vi "Dresden R2R Sputter 03.02.2018 IY24.vi"() -> ()   [LabVIEW 2009] (continued)
                                n28839 = case shown="False" w33825 {
                                frame #0 {
                                n28840 = local write "Pc_bv4_auto_set_pressure"(TRUE ("Pc_bv1_auto_set_pressure")) -> ()
                                }
                                frame #1 {
                                }
                                }
                                }
                                frame #1 {
                                }
                                }
                                }
                                frame #6 {
                                n28841 = local read "Semi"() -> (w33831:bool)
                                n28842 = case shown="False" w33831 {
                                frame #0 {
                                n28843 = while {
                                i -> [w33842]
                                stop <- w33833 stop-if-true
                                n28844 = local read "Set_pressure_value 4"() -> (w33837:dbl)
                                n28845 = Greater?(x=w33842, y=300) -> (0:w33835:bool)
                                n28846 = Add(x=1.0, y=w33837) -> (x+y=w33838:dbl)
                                n28847 = Subtract(x=w33837, y=1.0) -> (x-y=w33839:dbl)
                                n28848 = local read "Pressure 4"() -> (w33832:i32)
                                n28849 = In Range and Coerce(upper limit=w33838, x=w33832, lower limit=w33839) -> (In Range?=w33836:bool)  [unwired: 1 out]
                                n28850 = case shown="False" w33836 {
                                tunnel: [FALSE TRUE] -> w33834
                                frame #0 {
                                n28851 = Wait Until Next ms Multiple(millisecond multiple=u32 200) -> ()  [unwired: 1 out]
                                }
                                frame #1 {
                                }
                                }
                                n28852 = Or(x=w33834, y=w33835) -> (x .or. y?=w33833:bool)
                                }
                                }
                                frame #1 {
                                }
                                }
                                }
                                frame #7 {
                                n28853 = local read "Semi"() -> (w33847:bool)
                                n28854 = case shown="False" w33847 {
                                frame #0 {
                                n28855 = local read "Set_pressure_value 4"() -> (w33850:dbl)
                                n28856 = Add(x=1.0, y=w33850) -> (x+y=w33851:dbl)
                                n28857 = Subtract(x=w33850, y=1.0) -> (x-y=w33852:dbl)
                                n28858 = local read "Pressure 4"() -> (w33848:i32)
                                n28859 = In Range and Coerce(upper limit=w33851, x=w33848, lower limit=w33852) -> (In Range?=w33849:bool)  [unwired: 1 out]
                                n28860 = case shown="False" w33849 {
                                frame #0 {
                                n28861 = local write "Semi"(TRUE ("Semi")) -> ()
                                n28862 = local write "Error Message"("Coating Pressure could not be adjusted !" ("Error Message")) -> ()
                                }
                                frame #1 {
                                }
                                }
                                }
                                frame #1 {
                                }
                                }
                                }
                                }
                                }
                                frame #1 {
                                }
                                }
                                }
                                frame #1 {
                                n28863 = local read "Semi"() -> (w33857:bool)
                                n28864 = case shown="False" w33857 {
                                frame #0 {
                                n28865 = local write "SDC1 9"(TRUE ("SDC1 9")) -> ()
                                n28866 = Wait (ms)(milliseconds to wait=u32 1000) -> ()  [unwired: 1 out]
                                }
                                frame #1 {
                                }
                                }
                                }
                                }
                                }
                                }
                                }
                                frame #1 {
                                }
                                }
                                }
                                frame #11 {
                                n28867 = local read "Semi"() -> (w33860:bool)
                                n28868 = case shown="False" w33860 {
                                frame #0 {
                                n28869 = local write "Start_roll"(TRUE ("Start_roll")) -> ()
                                n28870 = Wait (ms)(milliseconds to wait=u32 300) -> ()  [unwired: 1 out]
                                }
                                frame #1 {
                                }
                                }
                                }
                                frame #12 {
                                n28871 = local read "Semi"() -> (w33863:bool)
                                n28872 = case shown="False" w33863 {
                                frame #0 {
                                n28873 = stacked-sequence {
                                frame #0 {
                                n28874 = local read "R Single RF Step1 Coating Power Active"() -> (w33864:bool)
                                n28875 = case shown="True" w33864 {
                                frame #0 {
                                }
                                frame #1 {
                                n28876 = while {
                                stop <- w33866 stop-if-true
                                n28877 = local read "R Single RF Interval length"() -> (w33870:dbl)
                                n28878 = local read "Actual Length"() -> (w33869:dbl)
                                n28879 = Greater Or Equal?(x=w33869, y=w33870) -> (x >= y?=w33868:bool)
                                n28880 = local read "Semi"() -> (w33867:bool)
                                n28881 = Or(x=w33868, y=w33867) -> (x .or. y?=w33866:bool)
                                n28882 = Wait Until Next ms Multiple(millisecond multiple=u32 300) -> ()  [unwired: 1 out]
                                }
                                }
                                }
                                }
                                frame #1 {
                                n28883 = local read "R Single RF Step2 Coating Power Active"() -> (w33871:bool)
                                n28884 = case shown="True" w33871 {
                                frame #0 {
                                }
                                frame #1 {
                                n28885 = stacked-sequence {
                                frame #0 {
                                n28886 = local read "Semi"() -> (w33872:bool)
                                n28887 = case shown="False" w33872 {
                                frame #0 {
                                n28888 = local read "R Single RF Step2 Coating Power"() -> (w33874:dbl)
                                n28889 = Wait (ms)(milliseconds to wait=u32 200) -> ()  [unwired: 1 out]
                                n28890 = local write "RF_forward_power_1"(w33874) -> ()
                                }
                                frame #1 {
                                }
                                }
                                }
                                frame #1 {
                                n28891 = local read "Semi"() -> (w33875:bool)
                                n28892 = case shown="False" w33875 {
                                frame #0 {
                                n28893 = local write "RF set auto"(TRUE ("Dc_auto_set")) -> ()
                                }
                                frame #1 {
                                }
                                }
                                }
                                frame #2 {
                                n28894 = while {
                                stop <- w33881 stop-if-true
                                n28895 = local read "R Single RF Interval length"() -> (w33880:dbl)
                                n28896 = local read "Actual Length"() -> (w33884:dbl)
                                n28897 = Multiply(x=w33880, y=2.0) -> (x*y=w33878:dbl)
                                n28898 = Greater Or Equal?(x=w33884, y=w33878) -> (x >= y?=w33883:bool)
                                n28899 = local read "Semi"() -> (w33882:bool)
                                n28900 = Or(x=w33883, y=w33882) -> (x .or. y?=w33881:bool)
                                n28901 = Wait Until Next ms Multiple(millisecond multiple=u32 300) -> ()  [unwired: 1 out]
                                }
                                }
                                }
                                }
                                }
                                }
                                frame #2 {
                                n28902 = local read "R Single RF Step3 Coating Power Active"() -> (w33885:bool)
                                n28903 = case shown="True" w33885 {
                                frame #0 {
                                }
                                frame #1 {
                                n28904 = stacked-sequence {
                                frame #0 {
                                n28905 = local read "Semi"() -> (w33886:bool)
                                n28906 = case shown="False" w33886 {
                                frame #0 {
                                n28907 = local read "R Single RF Step3 Coating Power"() -> (w33888:dbl)
                                n28908 = Wait (ms)(milliseconds to wait=u32 200) -> ()  [unwired: 1 out]
                                n28909 = local write "RF_forward_power_1"(w33888) -> ()
                                }
                                frame #1 {
                                }
                                }
                                }
                                frame #1 {
                                n28910 = local read "Semi"() -> (w33889:bool)
                                n28911 = case shown="False" w33889 {
                                frame #0 {
                                n28912 = local write "RF set auto"(TRUE ("Dc_auto_set")) -> ()
                                }
                                frame #1 {
                                }
                                }
                                }
                                frame #2 {
                                n28913 = while {
                                stop <- w33895 stop-if-true
                                n28914 = local read "R Single RF Interval length"() -> (w33894:dbl)
                                n28915 = local read "Actual Length"() -> (w33898:dbl)
                                n28916 = Multiply(x=w33894, y=3.0) -> (x*y=w33892:dbl)
                                n28917 = Greater Or Equal?(x=w33898, y=w33892) -> (x >= y?=w33897:bool)
                                n28918 = local read "Semi"() -> (w33896:bool)
                                n28919 = Or(x=w33897, y=w33896) -> (x .or. y?=w33895:bool)
                                n28920 = Wait Until Next ms Multiple(millisecond multiple=u32 300) -> ()  [unwired: 1 out]
                                }
                                }
                                }
                                }
                                }
                                }
                                frame #3 {
                                n28921 = local read "R Single RF Step4 Coating Power Active"() -> (w33899:bool)
                                n28922 = case shown="True" w33899 {
                                frame #0 {
                                }
                                frame #1 {
                                n28923 = stacked-sequence {
                                frame #0 {
                                n28924 = local read "Semi"() -> (w33900:bool)
                                n28925 = case shown="False" w33900 {
                                frame #0 {
                                n28926 = local read "R Single RF Step4 Coating Power"() -> (w33902:dbl)
                                n28927 = Wait (ms)(milliseconds to wait=u32 200) -> ()  [unwired: 1 out]
                                n28928 = local write "RF_forward_power_1"(w33902) -> ()
                                }
                                frame #1 {
                                }
                                }
                                }
                                frame #1 {
                                n28929 = local read "Semi"() -> (w33903:bool)
                                n28930 = case shown="False" w33903 {
                                frame #0 {
                                n28931 = local write "RF set auto"(TRUE ("Dc_auto_set")) -> ()
                                }
                                frame #1 {
                                }
                                }
                                }
                                frame #2 {
                                n28932 = while {
                                stop <- w33909 stop-if-true
                                n28933 = local read "R Single RF Interval length"() -> (w33908:dbl)
                                n28934 = local read "Actual Length"() -> (w33912:dbl)
                                n28935 = Multiply(x=w33908, y=4.0) -> (x*y=w33906:dbl)
                                n28936 = Greater Or Equal?(x=w33912, y=w33906) -> (x >= y?=w33911:bool)
                                n28937 = local read "Semi"() -> (w33910:bool)
                                n28938 = Or(x=w33911, y=w33910) -> (x .or. y?=w33909:bool)
                                n28939 = Wait Until Next ms Multiple(millisecond multiple=u32 300) -> ()  [unwired: 1 out]
                                }
                                }
                                }
                                }
                                }
                                }
                                frame #4 {
                                n28940 = local read "R Single RF Step5 Coating Power Active"() -> (w33913:bool)
                                n28941 = case shown="True" w33913 {
                                frame #0 {
                                }
                                frame #1 {
                                n28942 = stacked-sequence {
                                frame #0 {
                                n28943 = local read "Semi"() -> (w33914:bool)
                                n28944 = case shown="False" w33914 {
                                frame #0 {
                                n28945 = local read "R Single RF Step5 Coating Power"() -> (w33916:dbl)
                                n28946 = Wait (ms)(milliseconds to wait=u32 200) -> ()  [unwired: 1 out]
                                n28947 = local write "RF_forward_power_1"(w33916) -> ()
                                }
                                frame #1 {
                                }
                                }
                                }
                                frame #1 {
                                n28948 = local read "Semi"() -> (w33917:bool)
                                n28949 = case shown="False" w33917 {
                                frame #0 {
                                n28950 = local write "RF set auto"(TRUE ("Dc_auto_set")) -> ()
                                }
                                frame #1 {
                                }
                                }
                                }
                                frame #2 {
                                n28951 = while {
                                stop <- w33923 stop-if-true
                                n28952 = local read "R Single RF Interval length"() -> (w33922:dbl)
                                n28953 = local read "Actual Length"() -> (w33926:dbl)
                                n28954 = Multiply(x=w33922, y=5.0) -> (x*y=w33920:dbl)
                                n28955 = Greater Or Equal?(x=w33926, y=w33920) -> (x >= y?=w33925:bool)
                                n28956 = local read "Semi"() -> (w33924:bool)
                                n28957 = Or(x=w33925, y=w33924) -> (x .or. y?=w33923:bool)
                                n28958 = Wait Until Next ms Multiple(millisecond multiple=u32 300) -> ()  [unwired: 1 out]
                                }
                                }
                                }
                                }
                                }
                                }
                                }
                                }
                                frame #1 {
                                }
                                }
                                }
                                frame #13 {
                                n28959 = local read "Semi"() -> (w33927:bool)
                                n28960 = case shown="False" w33927 {
                                frame #0 {
                                n28961 = local write "SDC1 13b"(TRUE ("SDC1 13b")) -> ()
                                n28962 = Wait (ms)(milliseconds to wait=u32 1000) -> ()  [unwired: 1 out]
                                }
                                frame #1 {
                                }
                                }
                                }
                                }
                                }
                                frame #1 {
                                }
                                }
                                }
                                frame #17 {
                                # "encoder info  add to other web selection"
                                n28963 = stacked-sequence {
                                frame #0 {
                                n28964 = local read "Semi"() -> (w33930:bool)
                                n28965 = case shown="False" w33930 {
                                frame #0 {
                                # "salinim hareketi"
                                n28966 = local read "R_Web_selection"() -> (w33931:enum32{"Web", "Other"})
                                n28967 = case shown="\"Other\"" w33931 {
                                frame #0 {
                                # "TC -ROLL"
                                }
                                frame #1 {
                                n28968 = disable-structure shown="Disabled" {
                                frame #0 {
                                # "OTHER"
                                n28969 = local read "Semi"() -> (w33932:bool)
                                n28970 = case shown="False" w33932 {
                                frame #0 {
                                n28971 = stacked-sequence {
                                frame #0 {
                                n28972 = local read "Semi"() -> (w33933:bool)
                                n28973 = case shown="False" w33933 {
                                frame #0 {
                                n28974 = stacked-sequence {
                                frame #0 {
                                n28975 = local read "Semi"() -> (w33934:bool)
                                n28976 = case shown="False" w33934 {
                                frame #0 {
                                n28977 = while {
                                i -> [w33937]
                                stop <- w33938 stop-if-true
                                n28978 = Greater?(x=w33937, y=300) -> (0:w33935:bool)
                                n28979 = case shown="True" w33935 {
                                frame #0 {
                                }
                                frame #1 {
                                n28980 = local write "Semi"(TRUE ("Semi")) -> ()
                                }
                                }
                                n28981 = local read "RC_13"() -> (w33941:bool)
                                n28982 = case shown="False" w33941 {
                                tunnel: [FALSE ("ch2_1") TRUE ("ch2_1")] -> w33940
                                frame #0 {
                                n28983 = local write "Routine_check_transfer"(TRUE ("ch2_1")) -> ()
                                n28984 = Wait Until Next ms Multiple(millisecond multiple=u32 1000) -> ()  [unwired: 1 out]
                                }
                                frame #1 {
                                }
                                }
                                n28985 = local read "Semi"() -> (w33939:bool)
                                n28986 = Or(x=w33940, y=w33939) -> (x .or. y?=w33938:bool)
                                }
                                }
                                frame #1 {
                                }
                                }
                                }
                                frame #1 {
                                n28987 = local read "Semi"() -> (w33947:bool)
                                n28988 = case shown="False" w33947 {
                                frame #0 {
                                n28989 = while {
                                i -> [w33954]
                                stop <- w33949 stop-if-true
                                n28990 = Greater?(x=w33954, y=100) -> (0:w33952:bool)
                                n28991 = case shown="True" w33952 {
                                frame #0 {
                                }
                                frame #1 {
                                n28992 = local write "Error Message"("Transfer process was cancelled.\nPlease check GV connections." ("Error Message")) -> ()
                                n28993 = local write "Semi"(TRUE ("Semi")) -> ()
                                }
                                }
                                n28994 = local read "Ch1_Trns_interlock_di"() -> (w33948:bool)
                                n28995 = case shown="False" w33948 {
                                tunnel: [w33956 TRUE] -> w33951
                                frame #0 {
                                n28996 = local read "Ch1_TGV_control_di"() -> (w33955:bool)
                                n28997 = case shown="False" w33955 {
                                tunnel: [FALSE TRUE] -> w33956
                                frame #0 {
                                n28998 = Wait Until Next ms Multiple(millisecond multiple=u32 50) -> ()  [unwired: 1 out]
                                n28999 = local write "Ch1_TGV_control_do"(TRUE ("Ch1_pet_cool_up_do")) -> ()
                                }
                                frame #1 {
                                }
                                }
                                }
                                frame #1 {
                                }
                                }
                                n29000 = local read "Semi"() -> (w33950:bool)
                                n29001 = Or(x=w33951, y=w33950) -> (x .or. y?=w33949:bool)
                                }
                                }
                                frame #1 {
                                }
                                }
                                }
                                frame #2 {
                                n29002 = local read "Semi"() -> (w33964:bool)
                                n29003 = case shown="False" w33964 {
                                frame #0 {
                                n29004 = while {
                                i -> [w33971]
                                stop <- w33966 stop-if-true
                                n29005 = Greater?(x=w33971, y=100) -> (0:w33969:bool)
                                n29006 = case shown="True" w33969 {
                                frame #0 {
                                }
                                frame #1 {
                                n29007 = local write "Error Message"("Transfer process was cancelled.\nPlease check GV connections." ("Error Message")) -> ()
                                n29008 = local write "Semi"(TRUE ("Semi")) -> ()
                                }
                                }
                                n29009 = local read "Ch2_Trns_interlock_di"() -> (w33965:bool)
                                n29010 = case shown="False" w33965 {
                                tunnel: [w33973 TRUE] -> w33968
                                frame #0 {
                                n29011 = local read "Ch2_TGV_control_di"() -> (w33972:bool)
                                n29012 = case shown="False" w33972 {
                                tunnel: [FALSE TRUE] -> w33973
                                frame #0 {
                                n29013 = Wait Until Next ms Multiple(millisecond multiple=u32 50) -> ()  [unwired: 1 out]
                                n29014 = local write "Ch2_TGV_control_do"(TRUE ("Ch1_pet_cool_up_do")) -> ()
                                }
                                frame #1 {
                                }
                                }
                                }
                                frame #1 {
                                }
                                }
                                n29015 = local read "Semi"() -> (w33967:bool)
                                n29016 = Or(x=w33968, y=w33967) -> (x .or. y?=w33966:bool)
                                }
                                }
                                frame #1 {
                                }
                                }
                                }
                                frame #3 {
                                n29017 = local read "Semi"() -> (w33981:bool)
                                n29018 = case shown="False" w33981 {
                                frame #0 {
                                n29019 = while {
                                i -> [w33988]
                                stop <- w33983 stop-if-true
                                n29020 = Greater?(x=w33988, y=100) -> (0:w33986:bool)
                                n29021 = case shown="True" w33986 {
                                frame #0 {
                                }
                                frame #1 {
                                n29022 = local write "Error Message"("Transfer process was cancelled.\nPlease check GV connections." ("Error Message")) -> ()
                                n29023 = local write "Semi"(TRUE ("Semi")) -> ()
                                }
                                }
                                n29024 = local read "Ch3_Trns_interlock_di"() -> (w33982:bool)
                                n29025 = case shown="False" w33982 {
                                tunnel: [w33990 TRUE] -> w33985
                                frame #0 {
                                n29026 = local read "Ch3_TGV_control_di"() -> (w33989:bool)
                                n29027 = case shown="False" w33989 {
                                tunnel: [FALSE TRUE] -> w33990
                                frame #0 {
                                n29028 = Wait Until Next ms Multiple(millisecond multiple=u32 50) -> ()  [unwired: 1 out]
                                n29029 = local write "Ch3_TGV_control_do"(TRUE ("Ch1_pet_cool_up_do")) -> ()
                                }
                                frame #1 {
                                }
                                }
                                }
                                frame #1 {
                                }
                                }
                                n29030 = local read "Semi"() -> (w33984:bool)
                                n29031 = Or(x=w33985, y=w33984) -> (x .or. y?=w33983:bool)
                                }
                                }
                                frame #1 {
                                }
                                }
                                }
                                frame #4 {
                                n29032 = local read "Semi"() -> (w33998:bool)
                                n29033 = case shown="False" w33998 {
                                frame #0 {
                                n29034 = while {
                                i -> [w34005]
                                stop <- w34000 stop-if-true
                                n29035 = Greater?(x=w34005, y=100) -> (0:w34003:bool)
                                n29036 = case shown="True" w34003 {
                                frame #0 {
                                }
                                frame #1 {
                                n29037 = local write "Error Message"("Transfer process was cancelled.\nPlease check GV connections." ("Error Message")) -> ()
                                n29038 = local write "Semi"(TRUE ("Semi")) -> ()
                                }
                                }
                                n29039 = local read "Ch3_Trns_interlock_di"() -> (w33999:bool)
                                n29040 = case shown="False" w33999 {
                                tunnel: [w34007 TRUE] -> w34002
                                frame #0 {
                                n29041 = local read "Ch3_TGV_control_di"() -> (w34006:bool)
                                n29042 = case shown="False" w34006 {
                                tunnel: [FALSE TRUE] -> w34007
                                frame #0 {
                                n29043 = Wait Until Next ms Multiple(millisecond multiple=u32 50) -> ()  [unwired: 1 out]
                                n29044 = local write "Ch3_TGV_control_do"(TRUE ("Ch1_pet_cool_up_do")) -> ()
                                }
                                frame #1 {
                                }
                                }
                                }
                                frame #1 {
                                }
                                }
                                n29045 = local read "Semi"() -> (w34001:bool)
                                n29046 = Or(x=w34002, y=w34001) -> (x .or. y?=w34000:bool)
                                }
                                }
                                frame #1 {
                                }
                                }
                                }
                                frame #5 {
                                n29047 = local read "Semi"() -> (w34015:bool)
                                n29048 = case shown="False" w34015 {
                                frame #0 {
                                n29049 = while {
                                i -> [w34018]
                                stop <- w34019 stop-if-true
                                n29050 = Greater?(x=w34018, y=50) -> (0:w34016:bool)
                                n29051 = case shown="True" w34016 {
                                frame #0 {
                                }
                                frame #1 {
                                n29052 = local write "Error Message"("Transfer process was\ncancelled.Please check right slow sensor." ("Error Message")) -> ()
                                n29053 = local write "Semi"(TRUE ("Semi")) -> ()
                                }
                                }
                                n29054 = local read "Cnt_Right_slow_di"() -> (w34022:bool)
                                n29055 = case shown="False" w34022 {
                                tunnel: [FALSE ("Ch1_pet_cool_up_do") TRUE ("Ch1_pet_cool_up_do")] -> w34021
                                frame #0 {
                                n29056 = local write "Cnt_Right_slow_do"(TRUE ("Ch1_pet_cool_up_do")) -> ()
                                n29057 = Wait Until Next ms Multiple(millisecond multiple=u32 200) -> ()  [unwired: 1 out]
                                }
                                frame #1 {
                                }
                                }
                                n29058 = local read "Semi"() -> (w34020:bool)
                                n29059 = Or(x=w34021, y=w34020) -> (x .or. y?=w34019:bool)
                                }
                                }
                                frame #1 {
                                }
                                }
                                }
                                frame #6 {
                                n29060 = local read "Semi"() -> (w34029:bool)
                                n29061 = case shown="False" w34029 {
                                frame #0 {
                                n29062 = while {
                                i -> [w34030]
                                stop <- w34034 stop-if-true
                                n29063 = Greater?(x=w34030, y=50) -> (0:w34032:bool)
                                n29064 = case shown="True" w34032 {
                                frame #0 {
                                }
                                frame #1 {
                                n29065 = local write "Error Message"("Transfer process was\ncancelled.Please check right limit sensor." ("Error Message")) -> ()
                                n29066 = local write "Semi"(TRUE ("Semi")) -> ()
                                }
                                }
                                n29067 = local read "Cnt_Right_limit_di"() -> (w34036:bool)
                                n29068 = case shown="False" w34036 {
                                tunnel: [FALSE ("Ch1_pet_cool_up_do") TRUE ("Ch1_pet_cool_up_do")] -> w34035
                                frame #0 {
                                n29069 = local write "Cnt_Right_limit_do"(TRUE ("Ch1_pet_cool_up_do")) -> ()
                                n29070 = Wait Until Next ms Multiple(millisecond multiple=u32 200) -> ()  [unwired: 1 out]
                                }
                                frame #1 {
                                }
                                }
                                n29071 = local read "Semi"() -> (w34033:bool)
                                n29072 = Or(x=w34035, y=w34033) -> (x .or. y?=w34034:bool)
                                }
                                }
                                frame #1 {
                                }
                                }
                                }
                                frame #7 {
                                n29073 = local read "Semi"() -> (w34043:bool)
                                n29074 = case shown="False" w34043 {
                                frame #0 {
                                n29075 = while {
                                i -> [w34046]
                                stop <- w34047 stop-if-true
                                n29076 = Greater?(x=w34046, y=50) -> (0:w34044:bool)
                                n29077 = case shown="True" w34044 {
                                frame #0 {
                                }
                                frame #1 {
                                n29078 = local write "Error Message"("Transfer process was\ncancelled.Please check left slow sensor." ("Error Message")) -> ()
                                n29079 = local write "Semi"(TRUE ("Semi")) -> ()
                                }
                                }
                                n29080 = local read "Cnt_Left_slow_di"() -> (w34050:bool)
                                n29081 = case shown="False" w34050 {
                                tunnel: [FALSE ("Ch1_pet_cool_up_do") TRUE ("Ch1_pet_cool_up_do")] -> w34049
                                frame #0 {
                                n29082 = local write "Cnt_Left_slow_do"(TRUE ("Ch1_pet_cool_up_do")) -> ()
                                n29083 = Wait Until Next ms Multiple(millisecond multiple=u32 200) -> ()  [unwired: 1 out]
                                }
                                frame #1 {
                                }
                                }
                                n29084 = local read "Semi"() -> (w34048:bool)
                                n29085 = Or(x=w34049, y=w34048) -> (x .or. y?=w34047:bool)
                                }
                                }
                                frame #1 {
                                }
                                }
                                }
                                frame #8 {
                                n29086 = local read "Semi"() -> (w34057:bool)
                                n29087 = case shown="False" w34057 {
                                frame #0 {
                                n29088 = while {
                                i -> [w34058]
                                stop <- w34062 stop-if-true
                                n29089 = Greater?(x=w34058, y=50) -> (0:w34060:bool)
                                n29090 = case shown="True" w34060 {
                                frame #0 {
                                }
                                frame #1 {
                                n29091 = local write "Error Message"("Transfer process was\ncancelled.Please check left limit sensor." ("Error Message")) -> ()
                                n29092 = local write "Semi"(TRUE ("Semi")) -> ()
                                }
                                }
                                n29093 = local read "Cnt_Left_limit_di"() -> (w34064:bool)
                                n29094 = case shown="False" w34064 {
                                tunnel: [FALSE ("Ch1_pet_cool_up_do") TRUE ("Ch1_pet_cool_up_do")] -> w34063
                                frame #0 {
                                n29095 = local write "Cnt_Left_limit_do"(TRUE ("Ch1_pet_cool_up_do")) -> ()
                                n29096 = Wait Until Next ms Multiple(millisecond multiple=u32 200) -> ()  [unwired: 1 out]
                                }
                                frame #1 {
                                }
                                }
                                n29097 = local read "Semi"() -> (w34061:bool)
                                n29098 = Or(x=w34063, y=w34061) -> (x .or. y?=w34062:bool)
                                }
                                }
                                frame #1 {
                                }
                                }
                                }
                                }
                                }
                                frame #1 {
                                }
                                }
                                }
                                frame #1 {
                                n29099 = local read "Semi"() -> (w34071:bool)
                                n29100 = case shown="False" w34071 {
                                frame #0 {
                                n29101 = while {
                                i -> [w34077]
                                stop <- w34074 stop-if-true
                                n29102 = Greater?(x=w34077, y=50) -> (0:w34076:bool)
                                n29103 = case shown="True" w34076 {
                                frame #0 {
                                }
                                frame #1 {
                                n29104 = local write "Error Message"("" ("Error Message")) -> ()
                                n29105 = local write "Semi"(TRUE ("Semi")) -> ()
                                }
                                }
                                n29106 = local read "Casette_servo_start/stop_di"() -> (w34073:bool)
                                n29107 = case shown="False" w34073 {
                                tunnel: [FALSE TRUE] -> w34072
                                frame #0 {
                                n29108 = local write "Casette_servo_start/stop_do"(TRUE ("Casette_servo_left_direction_do")) -> ()
                                n29109 = Wait Until Next ms Multiple(millisecond multiple=u32 500) -> ()  [unwired: 1 out]
                                }
                                frame #1 {
                                }
                                }
                                n29110 = local read "Semi"() -> (w34075:bool)
                                n29111 = Or(x=w34072, y=w34075) -> (x .or. y?=w34074:bool)
                                }
                                }
                                frame #1 {
                                }
                                }
                                }
                                frame #2 {
                                n29112 = local read "Semi"() -> (w34085:bool)
                                n29113 = case shown="False" w34085 {
                                frame #0 {
                                n29114 = while {
                                i -> [w34091]
                                stop <- w34088 stop-if-true
                                n29115 = Greater?(x=w34091, y=50) -> (0:w34090:bool)
                                n29116 = case shown="True" w34090 {
                                frame #0 {
                                }
                                frame #1 {
                                n29117 = local write "Error Message"("" ("Error Message")) -> ()
                                n29118 = local write "Semi"(TRUE ("Semi")) -> ()
                                }
                                }
                                n29119 = local read "Casette_servo_left_direction_di"() -> (w34087:bool)
                                n29120 = case shown="False" w34087 {
                                tunnel: [FALSE TRUE] -> w34086
                                frame #0 {
                                n29121 = local write "Casette_servo_left_direction_do"(TRUE ("Casette_servo_left_direction_do")) -> ()
                                n29122 = Wait Until Next ms Multiple(millisecond multiple=u32 200) -> ()  [unwired: 1 out]
                                }
                                frame #1 {
                                }
                                }
                                n29123 = local read "Semi"() -> (w34089:bool)
                                n29124 = Or(x=w34086, y=w34089) -> (x .or. y?=w34088:bool)
                                }
                                }
                                frame #1 {
                                }
                                }
                                }
                                frame #3 {
                                # "casette motion"
                                n29125 = while {
                                i -> [w34101]
                                stop <- w34099 stop-if-true
                                n29126 = Greater?(x=w34101, y=200) -> (0:w34102:bool)
                                n29127 = case shown="True" w34102 {
                                frame #0 {
                                }
                                frame #1 {
                                n29128 = local write "Semi"(TRUE ("Semi")) -> ()
                                }
                                }
                                n29129 = local read "Counter_read_data"() -> (w34107:i16)
                                n29130 = Greater?(x=w34107, y=i16 0) -> (0:w34105:bool)
                                n29131 = case shown="True" w34105 {
                                tunnel: [TRUE TRUE] -> w34104
                                frame #0 {
                                }
                                frame #1 {
                                n29132 = local write "Casette_servo_start/stop_do"(FALSE ("Casette_servo_start/stop_do")) -> ()
                                n29133 = Wait Until Next ms Multiple(millisecond multiple=u32 200) -> ()  [unwired: 1 out]